vi "Pantallaperrona.vi"() -> ()   [LabVIEW 2020]
panel:
  in  "?":bool
  in  "?":bool
  in  "?":bool
  # "UNIDAD PROFESIONAL INTERDISCIPLINARIA DE INGENIERIAS CAMPUS ZACATECAS"
  # "PROYECTO INSTRUMENTACIÓN VIRTUAL"
  # "TERRARIO INTELIGENTE"
  # "Integrantes:"
  # "Teodoro Emiliano Noriega Gonzalez"
  # "Francisco Emiliano Romo Castañeda"
  # "Jorge Eduardo Hernández Esquivel"
  # "Grupo: 3MM3"
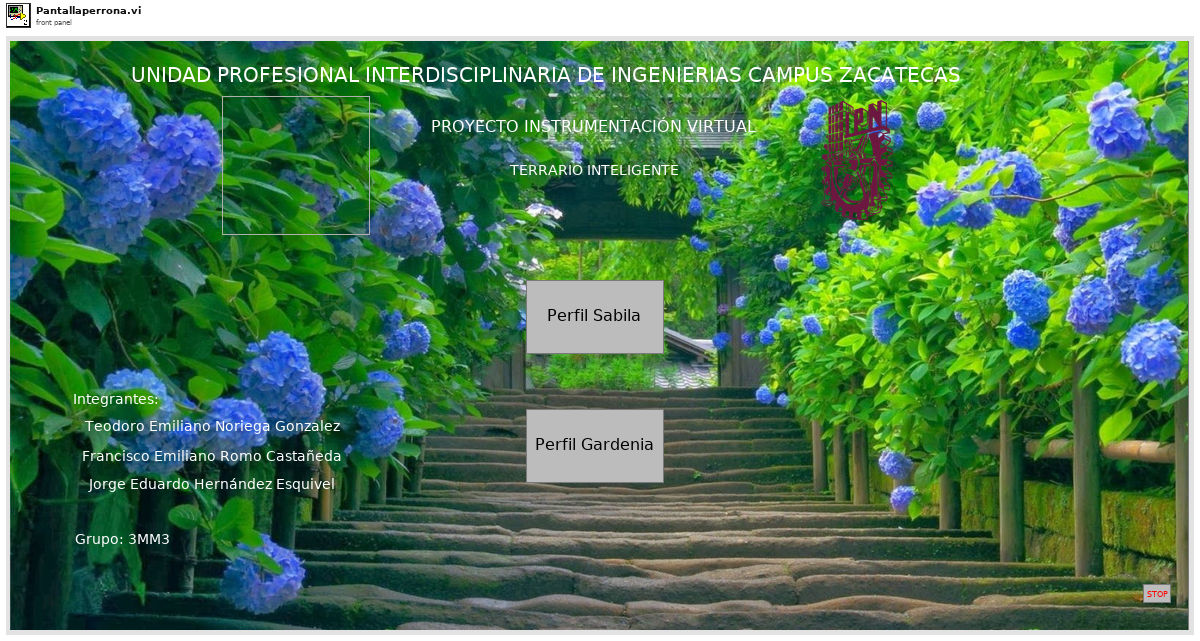
[diagram p1: front panel]
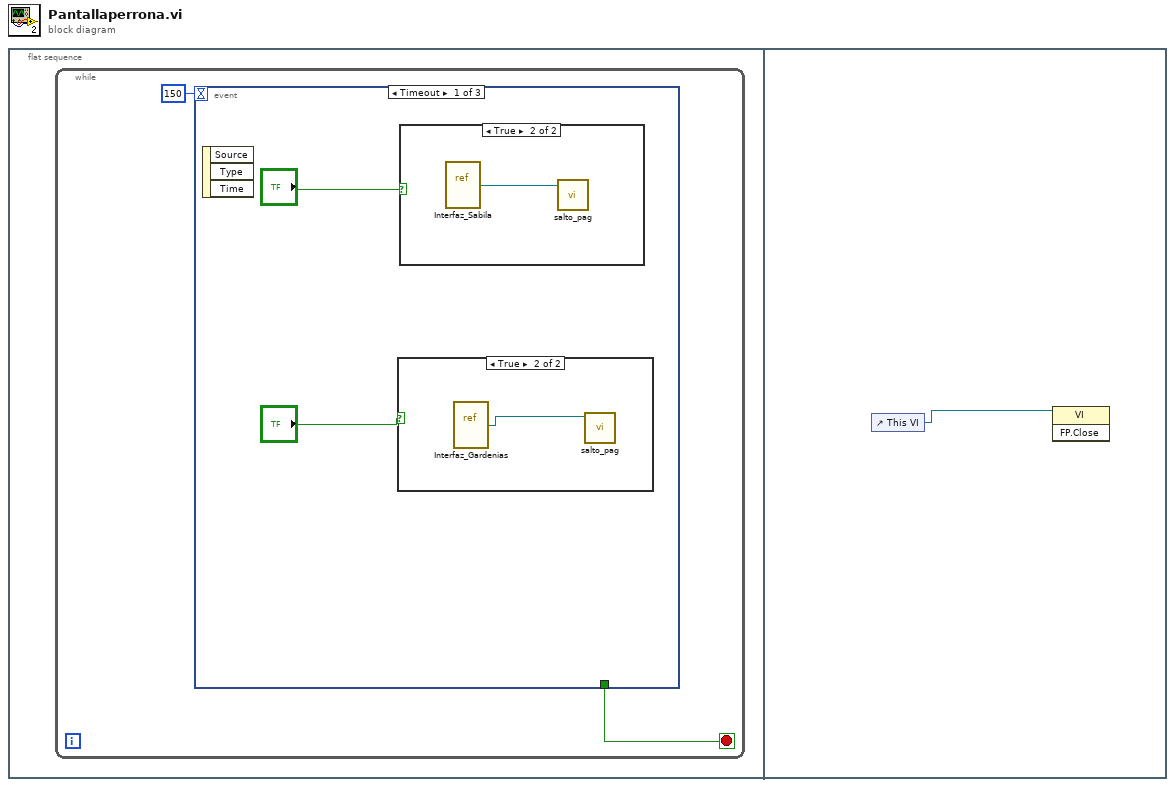
[diagram p0: block diagram]
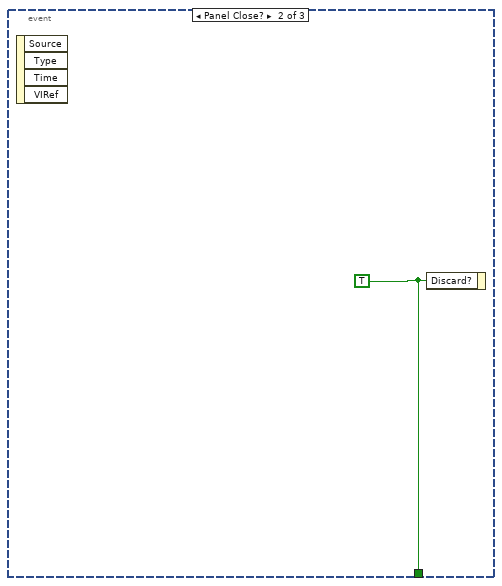
[diagram p4: hidden frame]
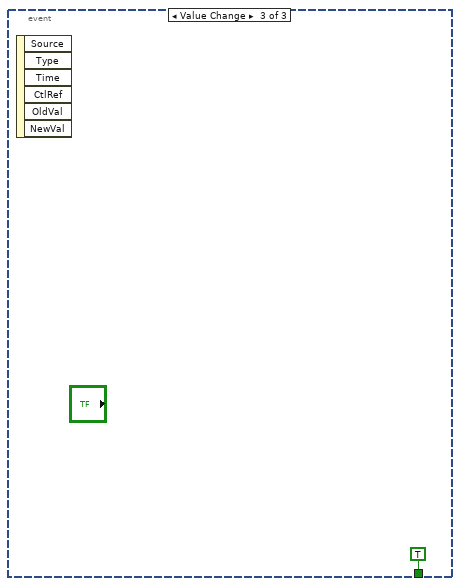
[diagram p5: hidden frame]
diagram:
  n1 = flat-sequence {
    frame #0 {
      n2 = while {
        stop <- w2 stop-if-true
        n3 = event shown="[0] Timeout" {
          selector: _ -> [_ _ _]
          dyn-events: _ -> [_ _ _]
          timeout: 150 -> [_ _ _]
          tunnel: [_ w7 TRUE ("Discard?")] -> w2
          event Timeout {
            n4 = event-data() -> ()  [unwired: 1 in, 3 out]
            n5 = case shown="True" "?" {
              frame False {
              }
              frame True {
                n6 = vi-ref "Interfaz_Gardenias.vi"() -> (w5:refnum<vi>)
                n7 = call "salto_pag.vi"("reference"=w5) -> ()  [unwired: 11 in]
              }
            }
            n8 = case shown="True" "?" {
              frame False {
              }
              frame True {
                n9 = vi-ref "Interfaz_Sabila.vi"() -> (w6:refnum<vi>)
                n10 = call "salto_pag.vi"("reference"=w6) -> ()  [unwired: 11 in]
              }
            }
          }
          event Panel Close? {
            w7 = TRUE ("Discard?")
            n11 = event-data() -> ()  [unwired: 1 in, 4 out]
            n12 = event-data("Discard?"=w7) -> ()  [unwired: 1 in, 1 out]
          }
          event Value Change {
            n13 = event-data() -> ()  [unwired: 1 in, 6 out]
          }
        }
      }
    }
    frame #1 {
      n14 = control-ref of="This VI"() -> (w9:refnum<vi>)
      n15 = invoke class="VI" method="FP.Close"(reference=w9) -> ()  [unwired: 2 in, 3 out]
    }
  }
